vi "UHR-Fleezers Control (host) - 10.8MV_trial1.vi"() -> ()   [LabVIEW 2010] (continued)
          tunnel: [w5184] -> w5138
          tunnel: w5137 -> [w5184]
          tunnel: w5138 -> [w5188]
          frame #0 {
            n1094 = local read "Green Laser ON/Interlacing"() -> (w5156:bool)
            n1095 = local read "Green laser mode"() -> (w5155:enum32{"Laser ON", "Laser OFF", "Interlace"})
            n1096 = local read "Green FB On/Off"() -> (w5154:bool)
          }
          frame #1 {
            n1097 = property on="Green FB On/Off" class="Bool (strict)"("Val(Sgnl)"=FALSE ("Value (Signaling)")) -> ()  [unwired: 2 in, 2 out]
          }
          frame #2 {
            n1098 = property on="Green Laser ON/Interlacing" class="Bool (strict)"("Val(Sgnl)"=TRUE ("Value (Signaling)")) -> ()  [unwired: 2 in, 2 out]
            n1099 = property on="Flip Green Filter" class="Bool (strict)"("Val(Sgnl)"=TRUE ("Value (Signaling)")) -> ()  [unwired: 2 in, 2 out]
            n1100 = property on="Green laser mode" class="RadioBtnsControl (strict)"("Val(Sgnl)"=enum32{"Laser ON", "Laser OFF", "Interlace"}."Laser ON" ("Value (Signaling)")) -> ()  [unwired: 2 in, 2 out]
          }
          frame #3 {
            n1101 = Wait (ms)(milliseconds to wait=u32 500) -> ()  [unwired: 1 out]
          }
          frame #4 {
            n1102 = property on="Confocal Image" class="Bool (strict)"("Val(Sgnl)"=TRUE ("Value (Signaling)")) -> ()  [unwired: 2 in, 2 out]
          }
          frame #5 {
            n1103 = Wait (ms)(milliseconds to wait=u32 2000) -> ()  [unwired: 1 out]
          }
          frame #6 {
            n1104 = while {
              stop <- w5182 stop-if-true
              n1105 = local read "Saving..."() -> (w5183:bool)
              n1106 = Not(x=w5183) -> (.not. x?=w5182:bool)
            }
          }
          frame #7 {
            n1107 = property on="Flip Green Filter" class="Bool (strict)"("Val(Sgnl)"=TRUE ("Value (Signaling)")) -> ()  [unwired: 2 in, 2 out]
            n1108 = property on="Green Laser ON/Interlacing" class="Bool (strict)"("Val(Sgnl)"=w5187) -> ()  [unwired: 2 in, 2 out]
            n1109 = property on="Green laser mode" class="RadioBtnsControl (strict)"("Val(Sgnl)"=w5186) -> ()  [unwired: 2 in, 2 out]
          }
          frame #8 {
            n1110 = property on="Green FB On/Off" class="Bool (strict)"("Val(Sgnl)"=w5188) -> ()  [unwired: 2 in, 2 out]
          }
        }
      }
      event "Stop All": Value Change {
        n1111 = event-data() -> ()  [unwired: 1 in, 5 out]
        n1112 = local read "Stop All"() -> (w5189:bool)
      }
    }
    n1113 = node-c288() -> ()  [unwired: 1 in, 1 out]
  }
  n1114 = node-c288() -> (w76:T26)  [unwired: 4 out]
  n1115 = timed-loop "Mouse control: trap position (AOM deflection), set confocal spot from image" {
    tunnel: [w5191] -> w34
    tunnel: w24 -> [w5190]
    timing: w76 -> [_]
    timing-out: [_] -> w75
    stop <- w5191 stop-if-true
    n1116 = node-c288() -> ()  [unwired: 2 out]
    n1117 = event shown="[0] \"Pane\": Mouse Down" {
      selector: _ -> [_ _]
      dyn-events: _ -> [_ _]
      timeout: _ -> [_ _]
      tunnel: w5190 -> [w5194 _]
      event Mouse Down {
        n1118 = event-data() -> ("Time"=w5196:u32, "Coords"=w5195:T7, "Button"=w5197:u16)  [unwired: 6 out]
        n1119 = case shown="1" w5197 {
          tunnel: w5196 -> [_ _ w5300]
          tunnel: w5195 -> [_ w5234 w5298]
          tunnel: w5194 -> [_ _ w5296]
          frame 0, Default {
          }
          frame 1 {
            n1120 = property on="APD 2" class="ImageControl"() -> ("Displayed Image Position"=w5204:cluster{"Left":i32, "Top":i32})  [unwired: 2 in, 2 out]
            n1121 = property on="APD 1" class="ImageControl"() -> ("Displayed Image Position"=w5233:cluster{"Left":i32, "Top":i32})  [unwired: 2 in, 2 out]
            n1122 = property on="Detection Laser X" class="ImageControl"() -> ("Displayed Image Position"=w5230:cluster{"Left":i32, "Top":i32})  [unwired: 2 in, 2 out]
            n1123 = property on="Detection Laser Y" class="ImageControl"() -> ("Displayed Image Position"=w5229:cluster{"Left":i32, "Top":i32})  [unwired: 2 in, 2 out]
            n1124 = property on="APD 2" class="ImageControl"() -> ("Displayed Image Size"=w5203:cluster{"Width":u32, "Height":u32})  [unwired: 2 in, 2 out]
            n1125 = property on="APD 1" class="ImageControl"() -> ("Displayed Image Size"=w5231:cluster{"Width":u32, "Height":u32})  [unwired: 2 in, 2 out]
            n1126 = property on="Detection Laser X" class="ImageControl"() -> ("Displayed Image Size"=w5232:cluster{"Width":u32, "Height":u32})  [unwired: 2 in, 2 out]
            n1127 = property on="Detection Laser Y" class="ImageControl"() -> ("Displayed Image Size"=w5228:cluster{"Width":u32, "Height":u32})  [unwired: 2 in, 2 out]
            n1128 = Unbundle By Name(w5203) -> ("Width"=w5200:u32, "Height"=w5199:u32)
            n1129 = Unbundle By Name(w5204) -> ("Left"=w5202:i32, "Top"=w5201:i32)
            n1130 = Unbundle By Name(w5231) -> ("Width"=w5225:u32, "Height"=w5224:u32)
            n1131 = Unbundle By Name(w5232) -> ("Width"=w5221:u32, "Height"=w5220:u32)
            n1132 = Unbundle By Name(w5228) -> ("Width"=w5217:u32, "Height"=w5216:u32)
            n1133 = Unbundle By Name(w5233) -> ("Left"=w5227:i32, "Top"=w5226:i32)
            n1134 = Unbundle By Name(w5230) -> ("Left"=w5223:i32, "Top"=w5222:i32)
            n1135 = Unbundle By Name(w5229) -> ("Left"=w5219:i32, "Top"=w5218:i32)
            n1136 = Bundle("Left"=w5202, "Top"=w5201, "Width"=w5200, "Height"=w5199) -> (w5198:T35)  [unwired: 1 in]
            n1137 = Bundle("Left"=w5227, "Top"=w5226, "Width"=w5225, "Height"=w5224) -> (w5215:T35)  [unwired: 1 in]
            n1138 = Bundle("Left"=w5223, "Top"=w5222, "Width"=w5221, "Height"=w5220) -> (w5214:T35)  [unwired: 1 in]
            n1139 = Bundle("Left"=w5219, "Top"=w5218, "Width"=w5217, "Height"=w5216) -> (w5213:T35)  [unwired: 1 in]
            n1140 = Build Cluster Array(w5198, w5215, w5214, w5213) -> (w5212:T36)
            n1141 = for {
              tunnel: w5234 -> [w5245]
              tunnel: w5212 -> [w5246] mode=indexing
              shift-right: [w5243] -> w5210
              shift-left: TRUE -> [w5244]
              shift-right: [w5242] -> w5208
              shift-left: _ -> [w5238]
              shift-right: [w5241] -> w5207
              shift-left: _ -> [w5237]
              shift-right: [w5240] -> w5206
              shift-left: _ -> [w5236]
              shift-right: [w5239] -> w5205
              shift-left: _ -> [w5235]
              n1142 = case shown="True" w5244 {
                selector: w5244 -> [w5251 _]
                tunnel: w5246 -> [_ w5260]
                tunnel: w5245 -> [_ w5258]
                tunnel: [w5251 w5256] -> w5243
                tunnel: [w5250 w5255] -> w5242
                tunnel: [w5249 w5254] -> w5241
                tunnel: [w5248 w5253] -> w5240
                tunnel: [w5247 w5252] -> w5239
                tunnel: w5238 -> [w5250 _]
                tunnel: w5237 -> [w5249 _]
                tunnel: w5236 -> [w5248 _]
                tunnel: w5235 -> [w5247 _]
                frame False {
                }
                frame True {
                  n1143 = Unbundle(w5260) -> (w5259:T35)
                  n1144 = call "isclickinwindow.vi"("Image Param"=w5259, "Point32"=w5258) -> ("4 Y"=w5252:i32, "3 Height"=w5253:i32, "2 X"=w5254:i32, "1 Width"=w5255:i32, "In image?"=w5257:bool)  [unwired: 1 in]
                  n1145 = Not(x=w5257) -> (.not. x?=w5256:bool)
                }
              }
            }
            n1146 = Not(x=w5210) -> (.not. x?=w5209:bool)
            n1147 = case shown="True" w5209 {
              tunnel: w5207 -> [_ w5273]
              tunnel: w5205 -> [_ w5272]
              tunnel: w5208 -> [_ w5271]
              tunnel: w5206 -> [_ w5270]
              frame False {
              }
              frame True {
                w5266 = FALSE ("Get Point")
                n1148 = local read "Scan lines (y)"() -> (w5275:u64)
                n1149 = local read "Actual MCL Inc (V)"() -> (w5267:dbl)
                n1150 = local read "Scan steps (MCL)"() -> (w5274:u64)
                n1151 = Divide "Y Pix/step"(x=w5270, y=w5275) -> (x/y=w5282:dbl)
                n1152 = Divide "Y V/pix"(x=w5267, y=w5282) -> (x/y=w5281:dbl)
                n1153 = Divide "Y half step offset"(x=w5267, y=2.0) -> (x/y=w5283:dbl)
                n1154 = Divide "X pix/step"(x=w5271, y=w5274) -> (x/y=w5280:dbl)
                n1155 = Negate(x=w5283) -> (-x=w5284:dbl)
                n1156 = local read "Initial Y"() -> (w5290:dbl)
                n1157 = Multiply(x=w5272, y=w5281) -> (x*y=w5291:dbl)
                n1158 = Divide "X half step offset"(x=w5267, y=2.0) -> (x/y=w5277:dbl)
                n1159 = Divide "X V/pix"(x=w5267, y=w5280) -> (x/y=w5279:dbl)
                n1160 = Multiply(x=w5267, y=w5274) -> (x*y=w5286:dbl)
                n1161 = Compound Arithmetic op=ADD(w5284, w5291, w5290) -> (w5268:dbl)
                "Pointer Y (V)" <- w5268
                n1162 = Multiply(x=w5279, y=w5273) -> (x*y=w5288:dbl)
                n1163 = Negate(x=w5277) -> (-x=w5276:dbl)
                n1164 = local read "Initial X"() -> (w5289:dbl)
                n1165 = Negate(x=w5288) -> (-x=w5287:dbl)
                n1166 = Compound Arithmetic op=ADD(w5276, w5286, w5289, w5287) -> (w5269:dbl)
                "Pointer X (V)" <- w5269
                n1167 = Or(x="Set X Only", y="Set Confocal Spot (X-Y)") -> (x .or. y?=w5262:bool)
                n1168 = Or(x="Set Confocal Spot (X-Y)", y="Set Y Only") -> (x .or. y?=w5261:bool)
                n1169 = case shown="True" w5262 {
                  tunnel: w5269 -> [_ w5292]
                  frame False {
                  }
                  frame True {
                    n1170 = property on="AO2" class="Slide (strict)"("Val(Sgnl)"=w5292) -> ()  [unwired: 2 in, 2 out]
                  }
                }
                n1171 = case shown="True" w5261 {
                  tunnel: w5268 -> [_ w5293]
                  frame False {
                  }
                  frame True {
                    n1172 = property on="AO1" class="Slide (strict)"("Val(Sgnl)"=w5293) -> ()  [unwired: 2 in, 2 out]
                  }
                }
                n1173 = local write "Set Confocal Spot (X-Y)"(w5266) -> ()
                n1174 = local write "Set X Only"(w5266) -> ()
                n1175 = local write "Set Y Only"(w5266) -> ()
              }
            }
          }
          frame 3 {
            n1176 = local read "BD 2 Frequency 1 (MHz)"() -> (w5294:dbl)
            n1177 = local read "BD 1 Frequency 1 (MHz)"() -> (w5295:dbl)
            n1178 = local write "Manipulating Trap"(TRUE ("Manipulating Trap")) -> ()
            n1179 = local write "Coords"(T7 {"Horizontal"=0, "Vertical"=0} ("Coords")) -> ()
            n1180 = while {
              tunnel: w5300 -> [w5305]
              tunnel: w5298 -> [w5304]
              tunnel: w5296 -> [w5303]
              tunnel: w5295 -> [w5302]
              tunnel: w5294 -> [w5301]
              stop <- w5306 stop-if-true
              n1181 = event shown="[0] \"Pane\": Mouse Move" {
                selector: _ -> [_ _]
                dyn-events: _ -> [_ _]
                timeout: _ -> [_ _]
                tunnel: ["Force Manip Abort" w5370] -> w5306
                tunnel: w5305 -> [w5313 _]
                tunnel: w5304 -> [w5311 _]
                tunnel: w5303 -> [w5310 _]
                tunnel: w5302 -> [w5309 _]
                tunnel: w5301 -> [w5308 _]
                event Mouse Move {
                  n1182 = event-data() -> ("Time"=w5314:u32, "Coords"=w5315:T7)  [unwired: 3 out]
                  n1183 = Less?(x=w5314, y=w5313) -> (x < y?=w5312:bool)
                  n1184 = case "Makes sure old motion events prior to mouse click aren't used" shown="False" w5312 {
                    tunnel: w5315 -> [w5357 _]
                    tunnel: w5311 -> [w5358 _]
                    tunnel: w5310 -> [w5335 _]
                    tunnel: w5309 -> [w5331 _]
                    tunnel: w5308 -> [w5330 _]
                    frame False {
                      n1185 = Subtract(x=w5357, y=w5358) -> (x-y=w5356:T7)
                      "Coords" <- w5356
                      n1186 = local read "Y RF Frequency Limits (MHz)"() -> (w5316:T16)
                      n1187 = To Double Precision Float(number=w5356) -> (double precision float=w5355:cluster{"Horizontal":dbl, "Vertical":dbl})
                      n1188 = Multiply(x=cluster{"Horizontal":dbl, "Vertical":dbl} {"Horizontal"=-1.0, "Vertical"=1.0}, y="Manipulation Scaling") -> (x*y=w5351:cluster{"Horizontal":dbl, "Vertical":dbl})
                      n1189 = local read "X RF Frequency Limits (MHz)"() -> (w5317:T16)
                      n1190 = Multiply(x=w5355, y=w5351) -> (x*y=w5353:cluster{"Horizontal":dbl, "Vertical":dbl})
                      n1191 = Unbundle By Name(w5353) -> ("Horizontal"=w5348:dbl, "Vertical"=w5352:dbl)
                      n1192 = Unbundle By Name(w5316) -> ("Maximum"=w5319:dbl, "Minimum"=w5318:dbl)
                      n1193 = Boolean To (0,1)(Boolean="Manip. X?") -> (0, 1=w5346:i16)
                      n1194 = Boolean To (0,1)(Boolean="Manip. Y?") -> (0, 1=w5343:i16)
                      n1195 = local read "BD 1 Frequency 2 (MHz)"() -> (w5333:dbl)
                      n1196 = Multiply(x=w5352, y=w5343) -> (x*y=w5345:dbl)
                      n1197 = Multiply(x=w5346, y=w5348) -> (x*y=w5349:dbl)
                      n1198 = local read "BD 2 Frequency 2 (MHz)"() -> (w5332:dbl)
                      n1199 = Unbundle By Name(w5317) -> ("Maximum"=w5321:dbl, "Minimum"=w5320:dbl)
                      n1200 = Add(x=w5330, y=w5345) -> (x+y=w5323:dbl)
                      n1201 = Add(x=w5331, y=w5349) -> (x+y=w5325:dbl)
                      n1202 = In Range and Coerce(upper limit=w5321, x=w5325, lower limit=w5320) -> (coerced(x)=w5324:dbl)  [unwired: 1 out]
                      n1203 = In Range and Coerce(upper limit=w5319, x=w5323, lower limit=w5318) -> (coerced(x)=w5322:dbl)  [unwired: 1 out]
                      n1204 = Subtract(x=w5324, y=w5333) -> (x-y=w5342:dbl)
                      n1205 = Subtract(x=w5322, y=w5332) -> (x-y=w5341:dbl)
                      n1206 = Square(x=w5342) -> (x^2=w5340:dbl)
                      n1207 = Square(x=w5341) -> (x^2=w5339:dbl)
                      n1208 = Add(x=w5340, y=w5339) -> (x+y=w5338:dbl)
                      n1209 = Square Root(x=w5338) -> (sqrt(x)=w5334:dbl)
                      n1210 = In Range and Coerce(upper limit="Limit Max (MHz)", x=w5334, lower limit="Limit Min (MHz)") -> (In Range?=w5327:bool)  [unwired: 1 out]
                      n1211 = Not(x="Limits Enable") -> (.not. x?=w5326:bool)
                      n1212 = Or(x=w5327, y=w5326) -> (x .or. y?=w5328:bool)
                      n1213 = case shown="True" w5328 {
                        tunnel: w5335 -> [_ w5368]
                        tunnel: w5334 -> [_ w5359]
                        tunnel: w5324 -> [_ w5366]
                        tunnel: w5333 -> [_ w5365]
                        tunnel: w5322 -> [_ w5364]
                        tunnel: w5332 -> [_ w5363]
                        tunnel: w5317 -> [_ w5361]
                        tunnel: w5316 -> [_ w5360]
                        frame False {
                        }
                        frame True {
                          n1214 = local read "BD 1 Frequency 3 (MHz)"() -> (w5367:dbl)
                          n1215 = local read "BD 2 Frequency 3 (MHz)"() -> (w5362:dbl)
                          n1216 = local write "Trap Delta (MHz)"(w5359) -> ()
                          n1217 = property on="Initial delta (MHz)" class="DigNum (strict)"("Val(Sgnl)"=w5359) -> ()  [unwired: 2 in, 2 out]
                          n1218 = call "set RF board frequency - interlace.vi"("Board 2 Frequency Limits"=w5360, "Board 1 Frequency Limits"=w5361, "FPGA VI Reference In"=w5368, "Board 2 Frequency 3 (MHz)"=w5362, "Board 1 Frequency 3 (MHz)"=w5367, "Board 2 Frequency 2 (MHz)"=w5363, "Board 2 Frequency 1 (MHz)"=w5364, "Board 1 Frequency 2 (MHz)"=w5365, "Board 1 Frequency 1  (MHz)"=w5366) -> ()  [unwired: 1 in, 2 out]
                          n1219 = local write "BD 2 Frequency 1 (MHz)"(w5364) -> ()
                          n1220 = local write "BD 1 Frequency 1 (MHz)"(w5366) -> ()
                        }
                      }
                    }
                    frame True {
                    }
                  }
                }
                event Mouse Up {
                  n1221 = event-data() -> ("Button"=w5369:u16)  [unwired: 8 out]
                  n1222 = case shown="3" w5369 {
                    tunnel: [FALSE TRUE] -> w5370
                    frame 0, Default {
                    }
                    frame 3 {
                      n1223 = local write "Manipulating Trap"(FALSE ("Manipulating Trap")) -> ()
                    }
                  }
                }
              }
            }
          }
        }
      }
      event Mouse Move {
        n1224 = event-data() -> ()  [unwired: 6 out]
      }
    }
    n1225 = local read "Stop All"() -> (w5191:bool)
    n1226 = node-c288() -> ()  [unwired: 2 out]
  }
  n1227 = node-c288(i64 1 ("Period"), 1 ("Processor")) -> (w164:T26)  [unwired: 2 out]
  n1228 = timed-loop "Acquire Data" {
    tunnel: w24 -> [w5628]
    tunnel: w40 -> [w5627]
    tunnel: [w5658] -> w33
    tunnel: [w5652] -> w32
    timing: w164 -> [_]
    timing-out: [_] -> w163
    tunnel: w59 -> [w5456]
    stop <- "Stop All" stop-if-true
    (unwired) u32 0 ("Number of Elements")
    w5443 = "NI_ChannelName" ("name")
    n1229 = node-c288() -> ()  [unwired: 2 out]
    n1230 = First Call?() -> (First Call?: T/F=w5409:bool)
    n1231 = Or(x="Reset", y=w5409) -> (x .or. y?=w5410:bool)
    n1232 = case "Reset data stream" shown="True" w5410 {
      tunnel: w5628 -> [w5746 w5754]
      tunnel: w5627 -> [w5745 w5753]
      tunnel: [w5746 w5748] -> w5623
      tunnel: [w5745 w5747] -> w5622
      frame False {
      }
      frame True {
        w5751 = TRUE ("AI to FIFO")
        n1233 = local write "Overflow (data lost)"(FALSE ("Overflow (data lost)")) -> ()
        n1234 = call "reset FPGA DMA.vi"("error in"=w5753, "FPGA VI Reference In"=w5754) -> ("error out"=w5749:errorcluster, "FPGA VI Reference Out"=w5750:T19)
        n1235 = xnode "Read/Write Control"("FPGA VI Reference In"=w5750, "error in"=w5749, "AI to FIFO"=w5751, "APD to FIFO"=w5751) -> ("FPGA VI Reference Out"=w5748:T19, "error out"=w5747:errorcluster)
      }
    }
    n1236 = Or(x="Start AOD Scan", y="Trap Raster Scan") -> (x .or. y?=w5573:bool)
    n1237 = case "Start AOM raster scan" shown="True" w5573 {
      tunnel: w5623 -> [w7354 w7364]
      tunnel: w5622 -> [w7353 w7363]
      tunnel: [w7354 w7357] -> w5621
      tunnel: [w7353 w7356] -> w5620
      frame False {
      }
      frame True {
        n1238 = case shown="True" "Restart DMA? (AOD)" {
          tunnel: [w7775 w7777] -> w7358
          tunnel: [w7774 w7776] -> w7359
          tunnel: w7364 -> [w7775 w7779]
          tunnel: w7363 -> [w7774 w7778]
          frame False {
          }
          frame True {
            n1239 = local write "Overflow (data lost)"(FALSE ("Overflow (data lost)")) -> ()
            n1240 = call "reset FPGA DMA.vi"("error in"=w7778, "FPGA VI Reference In"=w7779) -> ("error out"=w7776:errorcluster, "FPGA VI Reference Out"=w7777:T19)
          }
        }
        n1241 = local write "Trap Raster Scan"(FALSE ("Trap Raster Scan")) -> ()
        n1242 = case shown="False" "Move MCL Also?" {
          tunnel: w7359 -> [w7367 w7476]
          tunnel: w7358 -> [w7368 w7477]
          tunnel: [w7366 w7480] -> w7357
          tunnel: [w7365 w7479] -> w7356
          frame False {
            w7369 = TRUE ("AI to FIFO")
            n1243 = xnode "Read/Write Control"("FPGA VI Reference In"=w7368, "error in"=w7367, "AI to FIFO"=w7369, "APD to FIFO"=w7369, "Start scan"=w7369) -> ("FPGA VI Reference Out"=w7366:T19, "error out"=w7365:errorcluster)
          }
          frame True {
            w7473 = FALSE ("1D or 2D Scan?")
            w7478 = TRUE ("AI to FIFO")
            # "Count for MCL loop"
            # "N total cycles"
            # "N steps"
            # "V_int"
            n1244 = local read "Scan Range (nm)"() -> (w7455:dbl)
            n1245 = local read "Number of F/B Scans (AOD)"() -> (w7472:u16)
            n1246 = Sign(1:w7455) -> (0:w7454:dbl)
            n1247 = Compound Arithmetic op=MULTIPLY(w7455, "MCL Step Position Ratio", "MCL/AOM Scale Tweak") -> (w7459:dbl)
            n1248 = Negate(x=w7454) -> (-x=w7451:dbl)
            n1249 = Multiply(x=w7451, y="MCL Step Increment (V_int)") -> (x*y=w7453:dbl)
            n1250 = Divide(x=w7459, y="MCL X Cal (nm/V)") -> (x/y=w7465:dbl)
            n1251 = Multiply(x=32767.0 ("y"), y=w7465) -> (x*y=w7471:dbl)
            n1252 = local read "Total Counts (ticks)"() -> (w7456:u32)
            n1253 = local read "Cycles/step (AOD)"() -> (w7467:u64)
            n1254 = local read "Scan steps (AOD)"() -> (w7468:u64)
            n1255 = Divide(x=w7471, y=10.0) -> (x/y=w7464:dbl)
            n1256 = Divide(x=w7464, y="MCL Step Increment (V_int)") -> (x/y=w7462:dbl)
            n1257 = Absolute Value(x=w7462) -> (abs(x)=w7450:dbl)
            n1258 = Compound Arithmetic op=MULTIPLY(w7468, w7467, w7456) -> (w7463:u64)
            n1259 = local write "wait to reset values"(w7478) -> ()
            n1260 = local write "MCL Scanning"(w7478) -> ()
            n1261 = Divide(x=w7463, y=w7450) -> (x/y=w7460:dbl)
            "MCL Count" <- w7460
            n1262 = xnode "Read/Write Control"("FPGA VI Reference In"=w7477, "error in"=w7476, "Scan steps (MCL)"=w7450, "Number of scans (MCL)"=w7472, "Cycles per step (MCL)"=u64 1, "Scan freq.  increment (MCL)"=w7453, "1D or 2D Scan?"=w7473, "MCL Scan Axis"=w7473, "Cont. Scan (MCL)"=w7473, "MCL count"=w7460) -> ("FPGA VI Reference Out"=w7475:T19, "error out"=w7474:errorcluster)
            n1263 = xnode "Read/Write Control"("FPGA VI Reference In"=w7475, "error in"=w7474, "AI to FIFO"=w7478, "APD to FIFO"=w7478, "Start scan"=w7478, "Start scan (MCL)"=w7478) -> ("FPGA VI Reference Out"=w7480:T19, "error out"=w7479:errorcluster)
          }
        }
        "Raster Scanning..." <- TRUE ("Scanning...")
      }
    }
    n1264 = And(x="Save scans", y=w5573) -> (x .and. y?=w5619:bool)
    n1265 = Compound Arithmetic op=OR("Start MCL Scan", "Confocal Image", "Confocal Linescan") -> (w5571:bool)
    n1266 = And(x="Save Data (MCL)", y=w5571) -> (x .and. y?=w5618:bool)
    n1267 = case "Start MCL raster scan" shown="True" w5571 {
      tunnel: w5621 -> [w6631 w6646]
      tunnel: w5620 -> [w6630 w6645]
      tunnel: [w6631 w6641] -> w5378
      tunnel: [w6630 w6640] -> w5377
      tunnel: [FALSE w6639] -> w5604
      tunnel: "Start MCL Scan" -> [_ w6634]
      tunnel: "Confocal Image" -> [_ w6633]
      tunnel: "Confocal Linescan" -> [_ _]
      frame False {
      }
      frame True {
        w6639 = TRUE
        n1268 = case shown="True" "Restart DMA? (MCL)" {
          tunnel: [w6891 w6893] -> w6644
          tunnel: [w6890 w6892] -> w6643
          tunnel: w6646 -> [w6891 w6896]
          tunnel: w6645 -> [w6890 w6895]
          frame False {
          }
          frame True {
            n1269 = call "reset FPGA DMA.vi"("error in"=w6895, "FPGA VI Reference In"=w6896) -> ("error out"=w6892:errorcluster, "FPGA VI Reference Out"=w6893:T19)
            n1270 = local write "Overflow (data lost)"(FALSE ("Overflow (data lost)")) -> ()
          }
        }
        n1271 = case shown="False" w6634 {
          selector: w6634 -> [_ w6650]
          tunnel: w6633 -> [w6649 _]
          tunnel: [w6649 w6650] -> w6632
          frame False {
            n1272 = property on="2D or 1D Scan" class="Bool (strict)"("Val(Sgnl)"=w6649) -> ()  [unwired: 2 in, 2 out]
            n1273 = property on="Confocal Image" class="Bool (strict)"("Value"=FALSE ("Start Confocal Map")) -> ()  [unwired: 2 in, 2 out]
          }
          frame True {
          }
        }
        n1274 = local write "MCL Scanning"(w6639) -> ()
        n1275 = local read "AO1"() -> (w6636:dbl)
        n1276 = local read "AO2"() -> (w6635:dbl)
        n1277 = case shown="True" "Center Scan" {
          tunnel: w6644 -> [w6657 w6769]
          tunnel: w6643 -> [w6656 w6768]
          tunnel: [w6655 w6767] -> w6641
          tunnel: [w6654 w6766] -> w6640
          tunnel: [w6652 w6753] -> w6638
          tunnel: [w6651 w6752] -> w6637
          tunnel: w6636 -> [w6652 w6758]
          tunnel: w6635 -> [w6651 w6761]
          tunnel: w6632 -> [_ _]
          frame False {
            w6653 = TRUE ("AI to FIFO")
            n1278 = xnode "Read/Write Control"("FPGA VI Reference In"=w6657, "error in"=w6656, "AI to FIFO"=w6653, "APD to FIFO"=w6653, "Start scan (MCL)"=w6653) -> ("FPGA VI Reference Out"=w6655:T19, "error out"=w6654:errorcluster)
          }
          frame True {
            w6765 = TRUE ("AI to FIFO")
            n1279 = local read "Scan steps (MCL)"() -> (w6744:u64)
            n1280 = local read "Scan lines (y)"() -> (w6740:u64)
            n1281 = local read "Fast Scan Dir"() -> (w6751:bool)
            n1282 = local read "Actual MCL Inc (V)"() -> (w6741:dbl)
            n1283 = Decrement(x=w6740) -> (x-1=w6739:u64)
            n1284 = Decrement(x=w6744) -> (x-1=w6743:u64)
            n1285 = Multiply(x=w6741, y=w6739) -> (x*y=w6738:dbl)
            n1286 = Divide(x=w6738, y=2.0) -> (x/y=w6748:dbl)
            n1287 = Multiply(x=w6741, y=w6743) -> (x*y=w6742:dbl)
            n1288 = Divide(x=w6742, y=2.0) -> (x/y=w6747:dbl)
            n1289 = Select(t=w6747, s=w6751, f=w6748) -> (s? t:f=w6746:dbl)
            n1290 = Select(t=w6748, s=w6751, f=w6747) -> (s? t:f=w6750:dbl)
            n1291 = Subtract(x=w6758, y=w6750) -> (x-y=w6749:dbl)
            n1292 = Subtract(x=w6761, y=w6746) -> (x-y=w6745:dbl)
            n1293 = local read "2D or 1D Scan"() -> (w6763:bool)
            n1294 = Not(x=w6751) -> (.not. x?=w6757:bool)
            n1295 = Not(x=w6763) -> (.not. x?=w6759:bool)
            n1296 = And(x=w6751, y=w6759) -> (x .and. y?=w6760:bool)
            n1297 = And(x=w6759, y=w6757) -> (x .and. y?=w6762:bool)
            n1298 = Select(t=w6761, s=w6762, f=w6745) -> (s? t:f=w6752:dbl)
            n1299 = Select(t=w6758, s=w6760, f=w6749) -> (s? t:f=w6753:dbl)
            n1300 = call "Volt to I16.vi"("Voltage In"=w6753) -> ("I16 Voltage Out"=w6756:i16)
            n1301 = call "Volt to I16.vi"("Voltage In"=w6752) -> ("I16 Voltage Out"=w6755:i16)
            n1302 = xnode "Read/Write Control"("FPGA VI Reference In"=w6769, "error in"=w6768, "AI to FIFO"=w6765, "APD to FIFO"=w6765, "Start scan (MCL)"=w6765, "AO1"=w6756, "AO2"=w6755) -> ("FPGA VI Reference Out"=w6767:T19, "error out"=w6766:errorcluster)
          }
        }
        "Initial Y" <- w6638
        "Initial X" <- w6637
        "wait to reset values" <- w6639
      }
    }
    n1303 = local read "Trap Pos Elements/DMA read"() -> (w5452:u32)
    n1304 = local read "Trap AI Elements/DMA read"() -> (w5376:u32)
    n1305 = local read "APD Elements/DMA read"() -> (w5495:u32)
    n1306 = local read "Trap AI FIFO Depth"() -> (w5668:u32)
    n1307 = xnode "Invoke Method"("FPGA VI Reference In"=w5378, "error in"=w5377, "Number of Elements"=w5452, "Timeout (ms)"=-1) -> ("Data"=w5416:u16[], "Elements Remaining"=→"Trap Pos FIFO El Remaining":u32)  [unwired: 2 out]
    n1308 = xnode "Invoke Method"("FPGA VI Reference In"=w5378, "error in"=w5377, "Number of Elements"=w5376, "Timeout (ms)"=-1 ("Timeout")) -> ("FPGA VI Reference Out"=w5380:T19, "error out"=w5379:errorcluster, "Data"=w5375:i16[], "Elements Remaining"=w5381:u32)
    "Trap AI FIFO El. Rem." <- w5381
    n1309 = xnode "Get APD Data"("FPGA VI Reference In"=w5378, "error in"=w5377, "Number of Elements"=w5495, "Timeout (ms)"=-1) -> ("Data"=w5494:u32[], "Elements Remaining"=→"APD FIFO Elements Remaining":u32)  [unwired: 2 out]
    n1310 = Subtract(x=w5668, y=w5376) -> (x-y=w5667:u32)
    n1311 = Decimate 1D Array(w5416) -> (w5413:u16[], w5415:u16[], w5414:u16[])
    n1312 = Divide(x=w5381, y=w5667) -> (x/y=w5666:dbl)
    "Buffer Status" <- w5666
    n1313 = To Unsigned Long Integer(number=w5413) -> (unsigned 32bit integer=w5412:u32[])
    n1314 = Join Numbers(hi=w5415, lo=w5414) -> ((hi.lo)=w5411:u32[])
    n1315 = Equal?(x=w5666, y=1.0) -> (x = y?=w5664:bool)
    n1316 = Join Numbers(hi=w5412, lo=w5411) -> ((hi.lo)=w5405:u64[])
    n1317 = call "IR AOM word to freq - vec.vi"("Frequency Word In (double vec)"=w5405) -> ("Frequency Out"=w5451:dbl[])
    n1318 = case "Alert buffer overflow" shown="True" w5664 {
      frame False {
      }
      frame True {
        n1319 = call <vilib>:"Beep.vi"() -> ()  [unwired: 3 in, 9 out]
        "Overflow (data lost)" <- TRUE ("Overflow (data lost)")
      }
    }
    n1320 = Decimate 1D Array(w5451) -> (w5450:dbl[], w5449:dbl[])
    n1321 = Array Size(array=w5375) -> (size(s)=→"Waveform Chart":i32)
    n1322 = Build Array(w5450, w5449) -> (w5448:dbl[][])
    n1323 = local read "Trap Sets"() -> (w5532:u32)
    n1324 = case "Deinterlace trap data, average down PSD" shown="2" w5532 {
      tunnel: w5375 -> [w6926 w6991]
      tunnel: [w6923 w6988] -> w5525
      tunnel: [w6926 w6990] -> w5408
      tunnel: "Detector Type" -> [w6925 w6986]
      tunnel: [w6924 w6989] -> w5524
      tunnel: [w6922 w6987] -> w5639
      frame 1, Default {
        n1325 = Divide(x=w6926, y=3276.7) -> (x/y=w6927:dbl[])
        n1326 = Decimate 1D Array(w6927) -> (w6936:dbl[], w6935:dbl[], w6934:dbl[], w6933:dbl[], w6932:dbl[], w6931:dbl[], w6930:dbl[], w6929:dbl[])
        n1327 = case shown="\"IR-QPD + PSD + FB-QPD position\"" w6925 {
          tunnel: w6936 -> [w6960 w6985]
          tunnel: w6935 -> [w6959 w6984]
          tunnel: w6934 -> [w6944 w6962]
          tunnel: w6933 -> [w6945 w6972]
          tunnel: w6932 -> [w6958 w6983]
          tunnel: w6931 -> [w6957 w6982]
          tunnel: w6930 -> [w6941 w6963]
          tunnel: w6929 -> [w6940 w6961]
          tunnel: [w6939 w6969] -> w6924
          tunnel: [w6938 w6968] -> w6923
          tunnel: [w6937 w6967] -> w6922
          frame "IR-QPD + PSD + FB-QPD", Default {
            w6937 = 0  # Channel pattern
            n1328 = Divide(x=w6960, y=w6945) -> (x/y=w6947:dbl[])
            n1329 = Divide(x=w6959, y=w6945) -> (x/y=w6946:dbl[])
            n1330 = Divide(x=w6958, y=w6941) -> (x/y=w6943:dbl[])
            n1331 = Divide(x=w6957, y=w6940) -> (x/y=w6942:dbl[])
            n1332 = Build Array(w6947, w6946, w6945, w6944, w6943, w6942, w6941, w6940) -> (w6938:dbl[][])
            n1333 = Bundle("T1 Y", "T1 X", "T1 Sum", "FB Sum", "PSD Y", "PSD X", "PSD Y Sum", "PSD X Sum") -> (w6956:T44)  [unwired: 1 out]
            n1334 = Cluster To Array(cluster=w6956) -> (array=w6939:string[])
          }
          frame "IR-QPD + PSD + FB-QPD position" {
            w6967 = 3  # Channel pattern
            n1335 = Negate(x=w6963) -> (-x=w6964:dbl[])
            n1336 = Divide(x=w6985, y=w6972) -> (x/y=w6974:dbl[])
            n1337 = Divide(x=w6984, y=w6972) -> (x/y=w6973:dbl[])
            n1338 = Divide(x=w6983, y=w6963) -> (x/y=w6971:dbl[])
            n1339 = Divide(x=w6982, y=w6964) -> (x/y=w6970:dbl[])
            n1340 = Build Array(w6974, w6973, w6972, w6961, w6962, w6971, w6970, w6963) -> (w6968:dbl[][])
            n1341 = Bundle("T1 Y", "T1 X", "T1 Sum", "FB X", "FB Sum", "PSD Y", "PSD X", "PSD Y Sum") -> (w6981:T44)  [unwired: 1 out]
            n1342 = Cluster To Array(cluster=w6981) -> (array=w6969:string[])
          }
        }
      }
      frame 2 {
        n1343 = case shown="\"UCB Fleezers 052511\"" w6986 {
          tunnel: w6991 -> [w7053 w7120 w7148 w7255]
          tunnel: [w6992 w7112 w7143 w7186] -> w6990
          tunnel: [w7019 w7103 w7145 w7233] -> w6989
          tunnel: [w7018 w7067 w7122 w7200] -> w6988
          tunnel: [w7012 w7102 w7185 w7231] -> w6987
          frame "IR-QPD + PSD + FB-QPD", Default {
            w7012 = 1  # Channel pattern
            # "time average x2 the 4th signal and the 4 psd signals (detection laser)"
            # "deinterlace 3 signals from qpd"
            n1344 = Decimate 1D Array(w7053) -> (w7052:i16[], w7051:i16[], w7017:i16[], w7050:i16[], w7040:i16[], w7038:i16[], w7037:i16[], w7035:i16[])
            n1345 = call "downsample 1D array - double.vi"("Ave N"=2.0, "Array In"=w7040) -> ("Array Out"=w7039:dbl[])  [unwired: 1 out]
            n1346 = call "downsample 1D array - double.vi"("Ave N"=2.0, "Array In"=w7035) -> ("Array Out"=w7034:dbl[])  [unwired: 1 out]
            n1347 = call "downsample 1D array - double.vi"("Ave N"=2.0, "Array In"=w7037) -> ("Array Out"=w7036:dbl[])  [unwired: 1 out]
            n1348 = call "downsample 1D array - double.vi"("Ave N"=2.0, "Array In"=w7038) -> ("Array Out"=w7020:dbl[])  [unwired: 1 out]
            n1349 = Decimate 1D Array(w7052) -> (w7049:i16[], w7021:i16[])
            n1350 = Decimate 1D Array(w7051) -> (w7048:i16[], w7046:i16[])
            n1351 = Decimate 1D Array(w7050) -> (w7047:i16[], w7045:i16[])
            n1352 = Decimate 1D Array(w7017) -> (w7016:i16[], w7015:i16[])
            n1353 = Interleave 1D Arrays(w7049, w7048, w7047, w7021, w7046, w7045, w7016, w7015, w7039, w7020, w7036, w7034) -> (w7033:dbl[])
            n1354 = To Word Integer(number=w7033) -> (16bit integer=w6992:i16[])
            n1355 = Divide(x=w7033, y=3276.7) -> (x/y=w7032:dbl[])
            n1356 = Decimate 1D Array(w7032) -> (w7031:dbl[], w7030:dbl[], w7029:dbl[], w7028:dbl[], w7027:dbl[], w7026:dbl[], w7014:dbl[], w7013:dbl[], w7025:dbl[], w7024:dbl[], w7023:dbl[], w7022:dbl[])
            n1357 = Divide(x=w7031, y=w7029) -> (x/y=w6999:dbl[])
            n1358 = Divide(x=w7030, y=w7029) -> (x/y=w6998:dbl[])
            n1359 = Divide(x=w7028, y=w7026) -> (x/y=w6997:dbl[])
            n1360 = Divide(x=w7027, y=w7026) -> (x/y=w6996:dbl[])
            n1361 = Divide(x=w7025, y=w7023) -> (x/y=w6995:dbl[])
            n1362 = Divide(x=w7024, y=w7022) -> (x/y=w6994:dbl[])
            n1363 = Bundle("T1 Y", "T1 X", "T1 Sum", "T2 Y", "T2 X", "T2 Sum", "T1 FB Sum", "T2 FB Sum", "PSD Y", "PSD X", "PSD Y Sum", "PSD X Sum") -> (w7000:T45)  [unwired: 1 out]
            n1364 = Build Array(w6999, w6998, w7029, w6997, w6996, w7026, w7014, w7013, w6995, w6994, w7023, w7022) -> (w7018:dbl[][])
            n1365 = Cluster To Array(cluster=w7000) -> (array=w7019:string[])
          }
          frame "IR-QPD + PSD + FB-QPD X position" {
            w7102 = 2  # Channel pattern
            # "convert\nADC numbers\nto volts"
            # "time average x2 the 3 psd signals (detection laser)"
            # "deinterlace 3 signals from qpds"
            n1366 = Decimate 1D Array(w7120) -> (w7119:i16[], w7118:i16[], w7055:i16[], w7056:i16[], w7065:i16[], w7062:i16[], w7059:i16[], w7090:i16[])
            n1367 = Decimate 1D Array(w7119) -> (w7117:i16[], w7104:i16[])
            n1368 = call "downsample 1D array - I16.vi"("Ave N"=2.0, "Array In"=w7065) -> ("Array Out"=w7063:i16[])  [unwired: 1 in]
            n1369 = call "downsample 1D array - I16.vi"("Ave N"=2.0, "Array In"=w7062) -> ("Array Out"=w7060:i16[])  [unwired: 1 in]
            n1370 = Decimate 1D Array(w7118) -> (w7116:i16[], w7114:i16[])
            n1371 = Decimate 1D Array(w7056) -> (w7115:i16[], w7113:i16[])
            n1372 = Decimate 1D Array(w7090) -> (w7089:i16[], w7087:i16[])
            n1373 = Decimate 1D Array(w7055) -> (w7088:i16[], w7086:i16[])
            n1374 = call "downsample 1D array - I16.vi"("Ave N"=2.0, "Array In"=w7059) -> ("Array Out"=w7057:i16[])  [unwired: 1 in]
            n1375 = Interleave 1D Arrays(w7117, w7116, w7115, w7104, w7114, w7113, w7089, w7088, w7087, w7086, w7063, w7060, w7057) -> (w7112:i16[])
            n1376 = Divide(x=w7112, y=3276.7) -> (x/y=w7111:dbl[])
            n1377 = Decimate 1D Array(w7111) -> (w7110:dbl[], w7109:dbl[], w7108:dbl[], w7107:dbl[], w7106:dbl[], w7105:dbl[], w7078:dbl[], w7076:dbl[], w7075:dbl[], w7073:dbl[], w7072:dbl[], w7071:dbl[], w7068:dbl[])
            n1378 = Divide(x=w7110, y=w7108) -> (x/y=w7094:dbl[])
            n1379 = Divide(x=w7109, y=w7108) -> (x/y=w7093:dbl[])
            n1380 = Divide(x=w7107, y=w7105) -> (x/y=w7092:dbl[])
            n1381 = Divide(x=w7106, y=w7105) -> (x/y=w7091:dbl[])
            n1382 = Divide(x=w7078, y=w7076) -> (x/y=w7077:dbl[])
            n1383 = Divide(x=w7075, y=w7073) -> (x/y=w7074:dbl[])
            n1384 = Divide(x=w7072, y=w7068) -> (x/y=w7070:dbl[])
            n1385 = Negate(x=w7068) -> (-x=w7066:dbl[])
            n1386 = Divide(x=w7071, y=w7066) -> (x/y=w7069:dbl[])
            n1387 = Bundle("T1 Y", "T1 X", "T1 Sum", "T2 Y", "T2 X", "T2 Sum", "T1 FB X", "T1 FB Sum", "T2 FB X", "T2 FB Sum", "PSD Y", "PSD X", "PSD Y Sum") -> (w7095:T46)  [unwired: 1 out]
            n1388 = Build Array(w7094, w7093, w7108, w7092, w7091, w7105, w7077, w7076, w7074, w7073, w7070, w7069, w7068) -> (w7067:dbl[][])
            n1389 = Cluster To Array(cluster=w7095) -> (array=w7103:string[])
          }
          frame "UCB Fleezers 052511" {
            w7185 = 2  # Channel pattern
            n1390 = Decimate 1D Array(w7148) -> (w7183:i16[], w7182:i16[], w7147:i16[], w7146:i16[], w7140:i16[], w7137:i16[], w7136:i16[], w7135:i16[])
            n1391 = Decimate 1D Array(w7183) -> (w7181:i16[], w7166:i16[])
            n1392 = Decimate 1D Array(w7182) -> (w7180:i16[], w7178:i16[])
            n1393 = Decimate 1D Array(w7147) -> (w7179:i16[], w7177:i16[])
            n1394 = Decimate 1D Array(w7146) -> (w7142:i16[], w7141:i16[])
            n1395 = Decimate 1D Array(w7140) -> (w7139:i16[], w7138:i16[])
            n1396 = call "downsample 1D array - I16.vi"("Ave N"=2.0, "Array In"=w7137) -> ("Array Out"=w7134:i16[])  [unwired: 1 in]
            n1397 = call "downsample 1D array - I16.vi"("Ave N"=2.0, "Array In"=w7136) -> ("Array Out"=w7133:i16[])  [unwired: 1 in]
            n1398 = call "downsample 1D array - I16.vi"("Ave N"=2.0, "Array In"=w7135) -> ("Array Out"=w7132:i16[])  [unwired: 1 in]
            n1399 = Interleave 1D Arrays(w7181, w7180, w7179, w7166, w7178, w7177, w7142, w7139, w7141, w7138, w7134, w7133, w7132) -> (w7143:i16[])
            n1400 = Divide(x=w7143, y=3276.7) -> (x/y=w7173:dbl[])
            n1401 = Decimate 1D Array(w7173) -> (w7172:dbl[], w7171:dbl[], w7170:dbl[], w7169:dbl[], w7168:dbl[], w7167:dbl[], w7131:dbl[], w7129:dbl[], w7128:dbl[], w7126:dbl[], w7125:dbl[], w7124:dbl[], w7123:dbl[])
            n1402 = Divide(x=w7172, y=w7170) -> (x/y=w7153:dbl[])
            n1403 = Divide(x=w7171, y=w7170) -> (x/y=w7152:dbl[])
            n1404 = Divide(x=w7169, y=w7167) -> (x/y=w7151:dbl[])
            n1405 = Divide(x=w7168, y=w7167) -> (x/y=w7150:dbl[])
            n1406 = Divide(x=w7131, y=w7129) -> (x/y=w7130:dbl[])
            n1407 = Divide(x=w7128, y=w7126) -> (x/y=w7127:dbl[])
            n1408 = Bundle("T1 Y", "T1 X", "T1 Sum", "T2 Y", "T2 X", "T2 Sum", "T1 FB X", "T2 FB Sum", "T2 FB X", "T2 FB Sum", "PSD Y", "PSD X", "PSD Sum") -> (w7154:T46)  [unwired: 1 out]
            n1409 = Build Array(w7153, w7152, w7170, w7151, w7150, w7167, w7130, w7129, w7127, w7126, w7125, w7124, w7123) -> (w7122:dbl[][])
            n1410 = Cluster To Array(cluster=w7154) -> (array=w7145:string[])
          }
          frame "IR-QPD + PSD + FB-QPD XY positions" {
            w7231 = 4  # Channel pattern
            # "time average x2 the 3 psd signals (detection laser)"
            # "deinterlace 3 signals from qpds"
            n1411 = Decimate 1D Array(w7255) -> (w7254:i16[], w7253:i16[], w7232:i16[], w7252:i16[], w7198:i16[], w7244:i16[], w7243:i16[], w7220:i16[])
            n1412 = Decimate 1D Array "QPD Y"(w7254) -> (w7251:i16[], w7234:i16[])
            n1413 = call "downsample 1D array - double.vi"("Ave N"=2.0, "Array In"=w7244) -> ("Array Out"=w7219:dbl[])  [unwired: 1 out]
            n1414 = call "downsample 1D array - double.vi"("Ave N"=2.0, "Array In"=w7243) -> ("Array Out"=w7218:dbl[])  [unwired: 1 out]
            n1415 = Decimate 1D Array "Feedback Sum"(w7232) -> (w7216:i16[], w7214:i16[])
            n1416 = Decimate 1D Array "Feedback Y"(w7198) -> (w7197:i16[], w7196:i16[])
            n1417 = Decimate 1D Array "Feedback X"(w7220) -> (w7217:i16[], w7215:i16[])
            n1418 = Decimate 1D Array "QPD Sum"(w7252) -> (w7249:i16[], w7247:i16[])
            n1419 = Decimate 1D Array "QPD X"(w7253) -> (w7250:i16[], w7248:i16[])
            n1420 = Interleave 1D Arrays(w7251, w7250, w7249, w7234, w7248, w7247, w7197, w7217, w7216, w7196, w7215, w7214, w7219, w7218) -> (w7242:dbl[])
            n1421 = To Word Integer(number=w7242) -> (16bit integer=w7186:i16[])
            n1422 = Divide(x=w7242, y=3276.7) -> (x/y=w7241:dbl[])
            n1423 = Decimate 1D Array(w7241) -> (w7240:dbl[], w7239:dbl[], w7238:dbl[], w7237:dbl[], w7236:dbl[], w7235:dbl[], w7193:dbl[], w7207:dbl[], w7191:dbl[], w7192:dbl[], w7205:dbl[], w7189:dbl[], w7203:dbl[], w7201:dbl[])
            n1424 = Divide(x=w7240, y=w7238) -> (x/y=w7224:dbl[])
            n1425 = Divide(x=w7239, y=w7238) -> (x/y=w7223:dbl[])
            n1426 = Divide(x=w7237, y=w7235) -> (x/y=w7222:dbl[])
            n1427 = Divide(x=w7236, y=w7235) -> (x/y=w7221:dbl[])
            n1428 = Divide(x=w7193, y=w7191) -> (x/y=w7190:dbl[])
            n1429 = Divide(x=w7207, y=w7191) -> (x/y=w7206:dbl[])
            n1430 = Divide(x=w7192, y=w7189) -> (x/y=w7188:dbl[])
            n1431 = Divide(x=w7205, y=w7189) -> (x/y=w7204:dbl[])
            n1432 = Negate(x=w7201) -> (-x=w7199:dbl[])
            n1433 = Divide(x=w7203, y=w7199) -> (x/y=w7202:dbl[])
            n1434 = Bundle("T1 Y", "T1 X", "T1 Sum", "T2 Y", "T2 X", "T2 Sum", "T1 FB Y", "T1 FB X", "T1 FB Sum", "T2 FB Y", "T2 FB X", "T2 FB Sum", "PSD X", "PSD Y Sum") -> (w7187:T47)  [unwired: 1 out]
            n1435 = Build Array(w7224, w7223, w7238, w7222, w7221, w7235, w7190, w7206, w7191, w7188, w7204, w7189, w7202, w7201) -> (w7200:dbl[][])
            n1436 = Cluster To Array(cluster=w7187) -> (array=w7233:string[])
          }
        }
      }
    }
    "AI labels" <- w5524
    n1437 = Decimate 1D Array(w5494) -> (w5522:u32[], w5458:u32[])
    n1438 = local read "DMA Update Period (s)"() -> (w5533:dbl)
    n1439 = local read "BD 1 Frequency 2 (MHz)"() -> (w5400:dbl)
    n1440 = local read "BD 1 Frequency 1 (MHz)"() -> (w5401:dbl)
    n1441 = Build Array(w5522, w5458) -> (w5601:u32[][])
    n1442 = local read "Data Period (s)"() -> (w5507:dbl)
    n1443 = Decimate 1D Array(w5408) -> (w5431:i16[], w5430:i16[], w5428:i16[], w5427:i16[])  [unwired: 9 out]
    n1444 = To Double Precision Float(number=w5601) -> (double precision float=w5602:dbl[][])
    n1445 = local read "APD Integration Time (s)"() -> (w5471:dbl)
    n1446 = Divide(x=w5431, y=w5430) -> (x/y=w5432:dbl[])
    n1447 = Divide(x=w5428, y=w5427) -> (x/y=w5429:dbl[])
    n1448 = feedback #1(0.0) -> (w5445:dbl)
    n1449 = Add(x=w5533, y=w5445) -> (x+y=w5641:dbl)
    n1450 = feedback-in #1(w5641) -> ()
    n1451 = local read "AOM X Cal (nm/MHz)"() -> (w5398:dbl)
    n1452 = To Time Stamp(1:w5445) -> (0:w5444:timestamp)
    n1453 = Split 1D Array(array=w5432, index="N El. to Ave.") -> (second subarray=w5435:dbl[])  [unwired: 1 out]
    n1454 = Split 1D Array(array=w5429, index="N El. to Ave.") -> (second subarray=w5434:dbl[])  [unwired: 1 out]
    n1455 = local read "Trap X AI1 (DMA)"() -> (w5433:T13)
    n1456 = Multiply(x=w5507, y="Trap Disp. Downsample") -> (x*y=w5446:dbl)
    "Display Period (s)" <- w5446
    n1457 = Bundle("BD 1 Frequency 1 (MHz)"=w5401, "BD 1 Frequency 2 (MHz)"=w5400) -> (w5402:T48)  [unwired: 1 out]
    n1458 = for "Trap AI" {
      tunnel: [w6921] -> w5635 mode=indexing
      tunnel: w5444 -> [w6911]
      tunnel: "Trap Disp. Downsample" -> [w6919]
      tunnel: w5525 -> [w6917] mode=indexing
      tunnel: w5507 -> [w6916]
      tunnel: w5524 -> [w6915] mode=indexing
      tunnel: w5443 -> [w6914]
      tunnel: [w6913] -> w5482 mode=indexing
      tunnel: w5446 -> [w6912]
      n1459 = Bundle By Name("Y"=w6917, "dt"=w6916) -> (w6918:waveform(dbl))  [unwired: 1 out]
      n1460 = Set Waveform Attribute(5:w6915, 6:w6914, 7:w6918) -> (3:w6913:waveform(dbl))  [unwired: 1 in, 2 out]
      n1461 = call "downsample 1D array - double.vi"("Ave N"=w6919, "Array In"=w6917) -> ("Array Out"=w6920:dbl[])  [unwired: 1 out]
      n1462 = Bundle By Name(cluster=w6913, "t0"=w6911, "Y"=w6920, "dt"=w6912) -> (w6921:waveform(dbl))
    }
    n1463 = call <vilib>:"Mean.vi"("X"=w5434) -> ("mean"=w5422:dbl)  [unwired: 1 out]
    n1464 = call <vilib>:"Mean.vi"("X"=w5435) -> ("mean"=w5423:dbl)  [unwired: 1 out]
    n1465 = Cluster To Array(cluster=w5402) -> (array=w5399:dbl[])
    n1466 = Reciprocal(x=w5446) -> (1/x=→"Trap Disp. Freq. (Hz)":dbl)
    n1467 = local read "Data points/scans (MCL)"() -> (w5613:dbl)
    n1468 = To Fixed-Point(number=w5422) -> (fixed-point=w5420:fxp<+/-,16,1>)  [unwired: 1 in]
    n1469 = To Fixed-Point(number=w5423) -> (fixed-point=w5421:fxp<+/-,16,1>)  [unwired: 1 in]
    n1470 = Bundle("Trap 1 Pos.", "Trap 2 Pos.") -> (w5442:cluster{string, string})  [unwired: 1 out]
    n1471 = Bundle By Name(cluster=w5433, "Set 1"=w5421, "Set 2"=w5420) -> (→"Trap X AI1 (DMA)":T13)
    n1472 = Cluster To Array(cluster=w5442) -> (array=w5439:string[])
    n1473 = for "Trap Position" {
      tunnel: w5448 -> [w5898] mode=indexing
      tunnel: "Trap Disp. Downsample" -> [w5897]
      tunnel: w5446 -> [w5895]
      tunnel: w5444 -> [w5894]
      tunnel: w5443 -> [w5892]
      tunnel: w5439 -> [w5891] mode=indexing
      tunnel: [w5890] -> w5397 mode=indexing
      tunnel: w5399 -> [w5888] mode=indexing
      tunnel: w5398 -> [w5886]
      n1474 = call "downsample 1D array - double.vi"("Ave N"=w5897, "Array In"=w5898) -> ("Array Out"=w5896:dbl[])  [unwired: 1 out]
      n1475 = Subtract(x=w5896, y=w5888) -> (x-y=w5889:dbl[])
      n1476 = Multiply(x=w5886, y=w5889) -> (x*y=w5887:dbl[])
      n1477 = Bundle By Name("Y"=w5887, "dt"=w5895, "t0"=w5894) -> (w5893:waveform(dbl))  [unwired: 1 out]
      n1478 = Set Waveform Attribute(5:w5891, 6:w5892, 7:w5893) -> (3:w5890:waveform(dbl))  [unwired: 1 in, 2 out]
    }
    "Trap Positions" <- w5397
    n1479 = Bundle("APD 1", "APD 2") -> (w5634:cluster{string, string})  [unwired: 1 out]
    n1480 = Cluster To Array(cluster=w5634) -> (array=w5631:string[])
    n1481 = for "APD" {
      tunnel: w5602 -> [w6900] mode=indexing
      tunnel: w5471 -> [w6908]
      tunnel: [w6904] -> w5478 mode=indexing
      tunnel: "APD Disp. Scale" -> [w6905]
      tunnel: w5443 -> [w6903]
      tunnel: w5631 -> [w6902] mode=indexing
      tunnel: "APD Disp. Downsample" -> [w6898]
      tunnel: [w6901] -> w5630
      tunnel: w5444 -> [w6897]
      n1482 = call "integrate 1D array interval - double.vi"("Ave N"=w6898, "Array In"=w6900) -> ("Array Out"=w6899:dbl[])  [unwired: 1 out]
      n1483 = Multiply(x=w6908, y=w6898) -> (x*y=w6901:dbl)
      n1484 = Divide(x=w6899, y=w6905) -> (x/y=w6906:dbl[])
      n1485 = Bundle By Name("t0"=w6897, "Y"=w6906, "dt"=w6901) -> (w6907:waveform(dbl))  [unwired: 1 out]
      n1486 = Set Waveform Attribute(5:w6902, 6:w6903, 7:w6907) -> (3:w6904:waveform(dbl))  [unwired: 1 in, 2 out]
    }
    "APD Display Period (s)" <- w5630
    n1487 = Reciprocal(x=w5630) -> (1/x=→"APD Display Freq. (Hz)":dbl)
    n1488 = local read "Display Period (s)"() -> (w5506:dbl)
    n1489 = Increment(x=w5613) -> (x+1=w5614:dbl)
    n1490 = Index Array(array=w5397, index=0) -> (element=w5395:waveform(dbl))
    n1491 = To Double Precision Float(number=w5522) -> (double precision float=w5521:dbl[])
    n1492 = feedback #2(w5614) -> (w5617:dbl)
    n1493 = Select(t=0, s=w5604, f=w5617) -> (s? t:f=w5610:dbl)
    n1494 = Array Size(array=w5521) -> (size(s)=w5616:i32)
    n1495 = Add(x=w5616, y=w5610) -> (x+y=w5611:dbl)
    n1496 = Unbundle By Name(w5395) -> ("Y"=w5393:dbl[])
    n1497 = feedback #3(w5522) -> (w5600:u32[])
    n1498 = Build Array (concatenate)(w5600, w5522) -> (w5597:u32[])
    n1499 = feedback #4(w5458) -> (w5477:u32[])
    n1500 = Divide(x="Bead Sep. Int. Time (s)", y=w5506) -> (x/y=w5391:dbl)
    n1501 = Build Array (concatenate)(w5477, w5458) -> (w5476:u32[])
    n1502 = Greater?(x=w5611, y=w5613) -> (0:w5612:bool)
    n1503 = feedback #5(w5393) -> (w5394:dbl[])
    n1504 = Build Array (concatenate)(w5393, w5394) -> (w5392:dbl[])
    n1505 = Select(t=w5610, s=w5612, f=w5611) -> (s? t:f=w5609:dbl)
    n1506 = feedback-in #2(w5609) -> ()
    n1507 = Array Size(array=w5597) -> (size(s)=w5594:i32)
    n1508 = Array Size(array=w5522) -> (size(s)=w5596:i32)
    n1509 = local read "MCL Scanning"() -> (w5607:bool)
    n1510 = local read "APD Integration Time (s)"() -> (w5485:dbl)
    n1511 = Build Array (concatenate)(w5478, w5635) -> (w5480:waveform(dbl)[])
    "All Signals" <- w5480
    n1512 = Split 1D Array(array=w5392, index=w5391) -> (first subarray=w5385:dbl[])  [unwired: 1 out]
    n1513 = feedback-in #5(w5385) -> ()
    n1514 = Multiply(x=w5596, y="APD Ave N") -> (x*y=w5595:dbl)
    n1515 = Greater?(x=w5594, y=w5595) -> (0:w5598:bool)
    n1516 = Not(x=w5612) -> (.not. x?=w5606:bool)
    n1517 = To Double Precision Float(number=w5458) -> (double precision float=w5457:dbl[])
    n1518 = call <vilib>:"Mean.vi"("X"=w5385) -> ("mean"=w5384:dbl)  [unwired: 1 out]
    "Mean T1 Position (nm)" <- w5384
    n1519 = Subtract(x=w5385, y=w5384) -> (x-y=w5390:dbl[])
    n1520 = Square(x=w5390) -> (x^2=w5389:dbl[])
    n1521 = And(x=w5606, y=w5607) -> (x .and. y?=w5608:bool)
    n1522 = call <vilib>:"Mean.vi"("X"=w5389) -> ("mean"=w5388:dbl)  [unwired: 1 out]
    n1523 = case shown="True" w5598 {
      tunnel: w5597 -> [w6481 w6488]
      tunnel: [w6481 w6486] -> w5538
      tunnel: w5595 -> [_ w6483]
      tunnel: w5594 -> [_ w6487]
      tunnel: w5476 -> [w6480 w6485]
      tunnel: [w6480 w6482] -> w5473
      frame False {
      }
      frame True {
        n1524 = Subtract(x=w6487, y=w6483) -> (x-y=w6484:dbl)
        n1525 = Array Subset(array=w6488, index=w6484, length=w6483) -> (w6486:u32[])
        n1526 = Array Subset(array=w6485, index=w6484, length=w6483) -> (w6482:u32[])
      }
    }
    n1527 = feedback-in #3(w5538) -> ()
    n1528 = feedback-in #4(w5473) -> ()